vi "期末專題_PlantFactory Eleccost Calculator.vi"() -> ()   [LabVIEW 2014]
panel:
  in  "PlantFactory Eleccost Calculator":T1
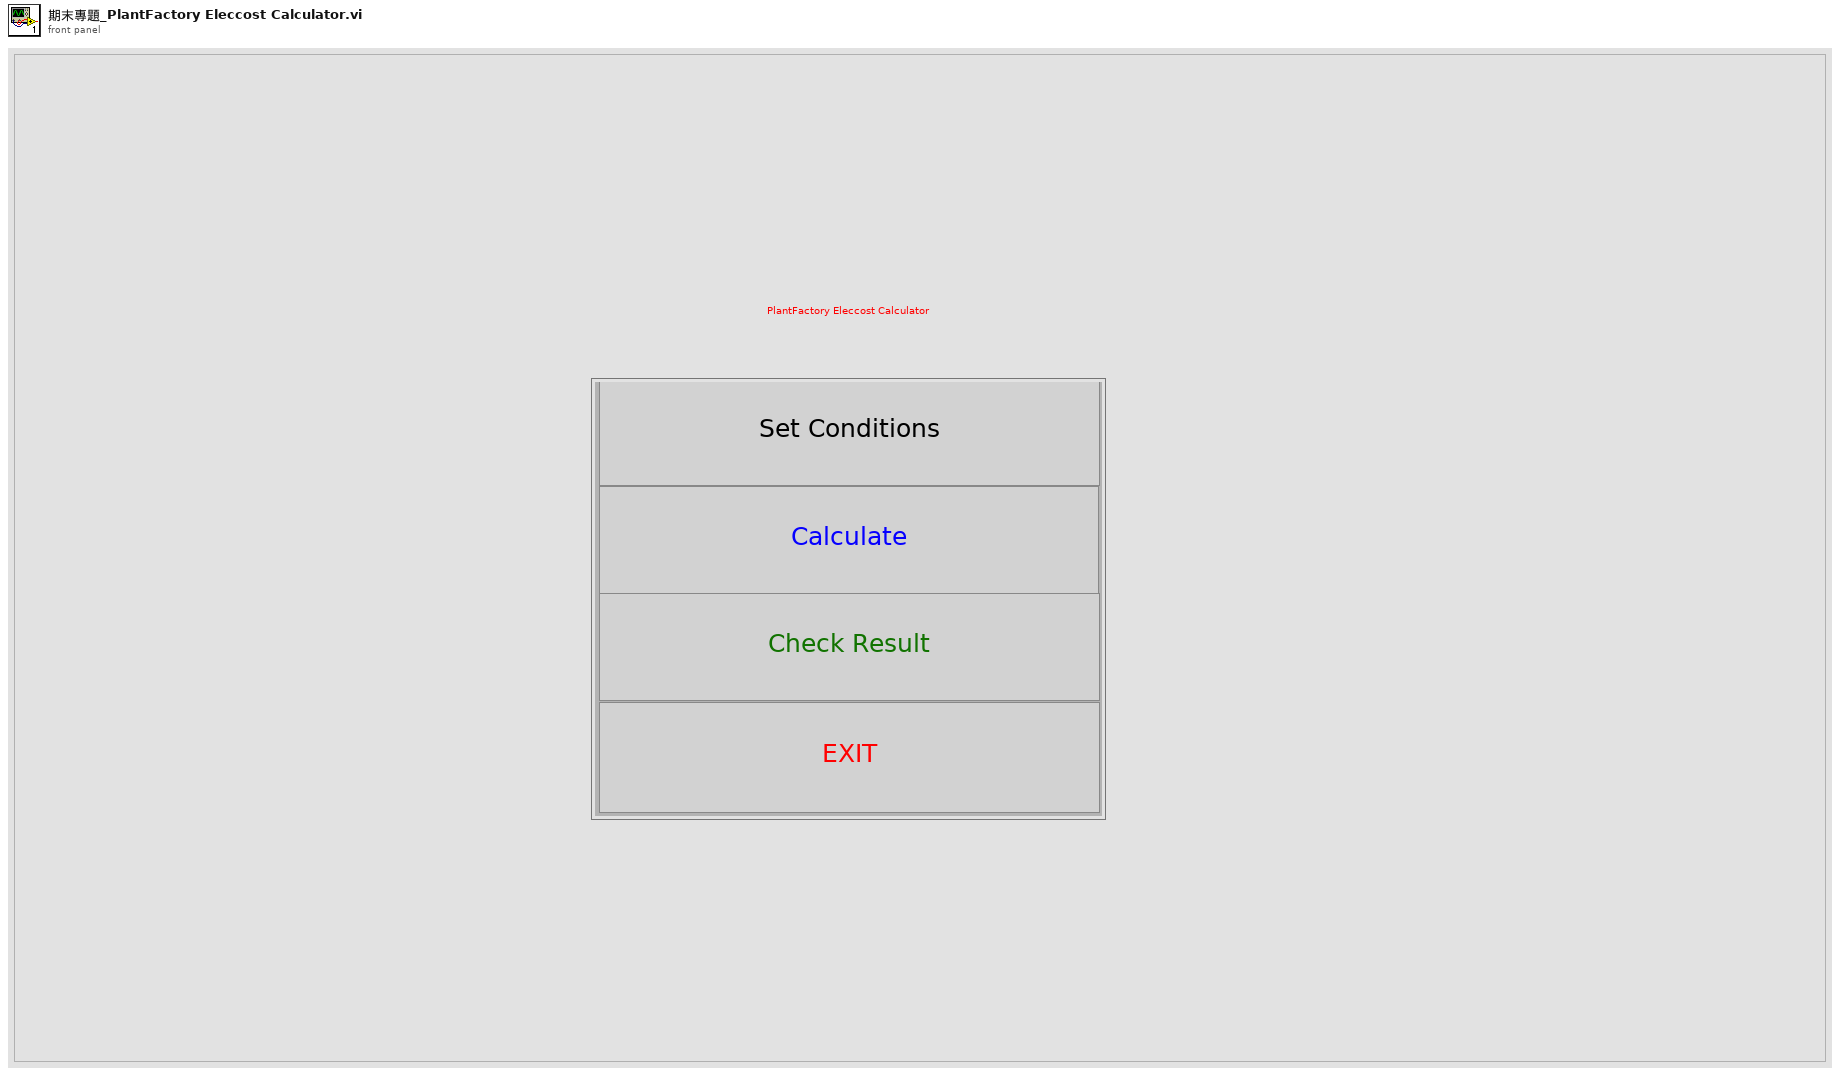
[diagram p1: front panel]
types:
  T1 = cluster{"set condi":bool, "calcu":bool, "outcome":bool, "exit":bool}
  T2 = cluster{"group Outcome":cluster{"Lightening Schedule":bool[], "group hourly total elecFee":dbl[], "group Total elecFee":dbl, "group hourly ACs elecFee":dbl[], "group ACs elecFee":dbl, "group hourly LEDs elecFee":dbl[], "group Total LEDs elecFee":dbl}, "group Outcome 2":cluster{"Lightening Schedule":bool[], "group hourly total elecFee":dbl[], "group Total elecFee":dbl, "group hourly ACs elecFee":dbl[], "group ACs elecFee":dbl, "group hourly LEDs elecFee":dbl[], "group Total LEDs elecFee":dbl}, "group Outcome 3":cluster{"Lightening Schedule":bool[], "group hourly total elecFee":dbl[], "group Total elecFee":dbl, "group hourly ACs elecFee":dbl[], "group ACs elecFee":dbl, "group hourly LEDs elecFee":dbl[], "group Total LEDs elecFee":dbl}, "Total elecFee":dbl}[]
  T3 = cluster{"input COP of ACs":dbl, "input setDay Temp":dbl, "input setNight Temp.":dbl}
  T4 = enum16{"wait button pressed", "init", "set conditions", "calcu", " outcome display"}
  T5 = enum8{"Enabled", "Disabled", "Disabled and Grayed Out"}
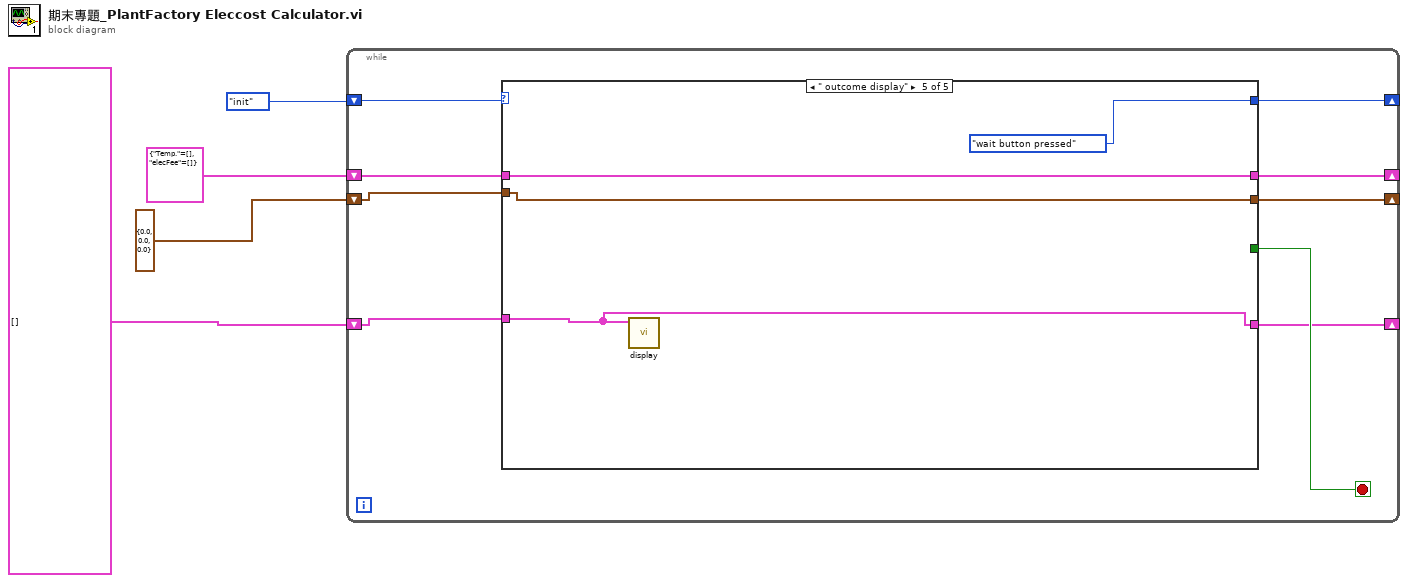
[diagram p0: block diagram]
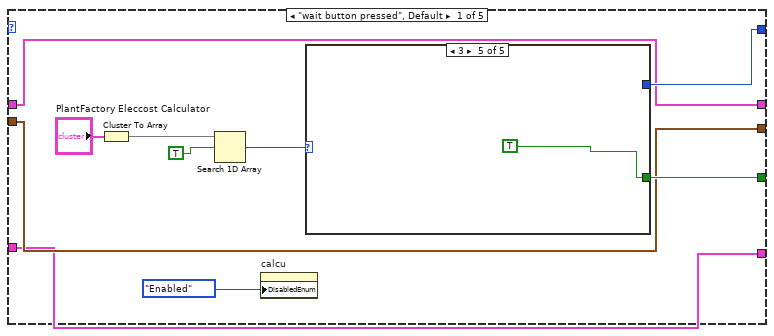
[diagram p2: hidden frame]
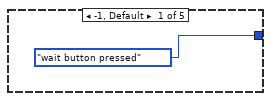
[diagram p3: hidden frame]
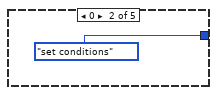
[diagram p4: hidden frame]
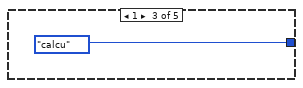
[diagram p5: hidden frame]
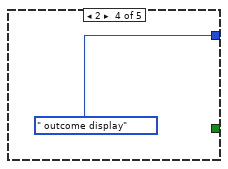
[diagram p6: hidden frame]
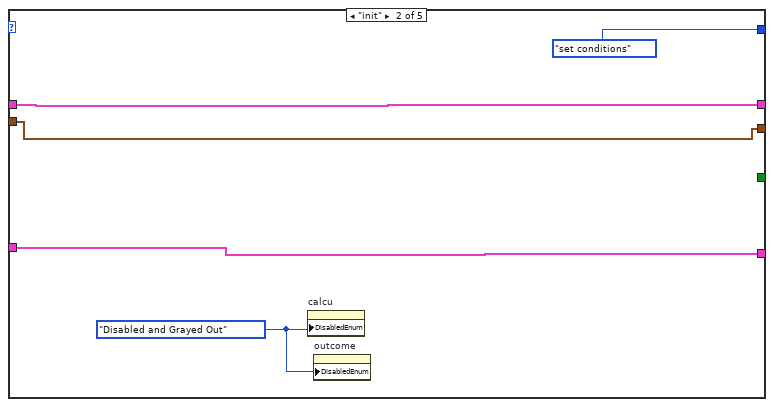
[diagram p7: hidden frame]
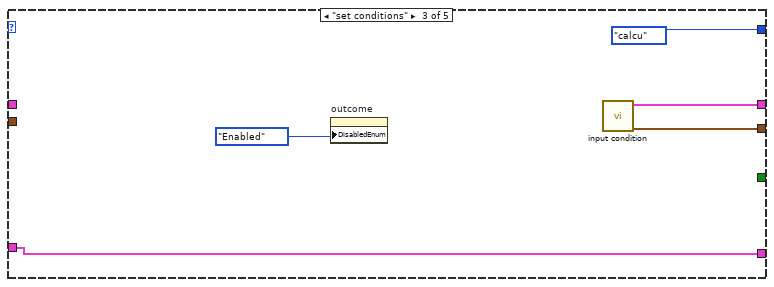
[diagram p8: hidden frame]
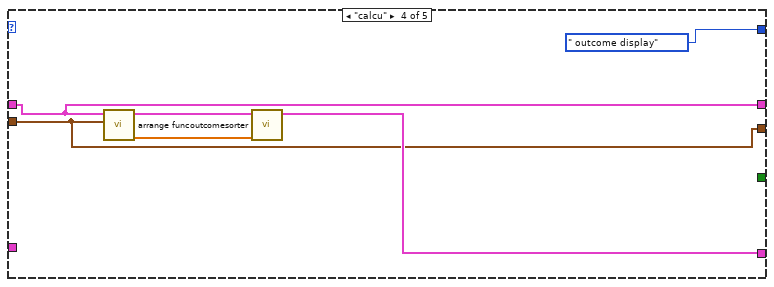
[diagram p9: hidden frame]
diagram:
  n1 = while {
    shift-right: [w13] -> _
    shift-left: T4."init" -> [w12]
    shift-right: [w10] -> _
    shift-left: cluster{"Temp.":dbl[], "elecFee":dbl[]} {"Temp."=[], "elecFee"=[]} ("input envTemp. & elecFee 2") -> [w7]
    shift-right: [w9] -> _
    shift-left: T3 {"input COP of ACs"=0.0, "input setDay Temp"=0.0, "input setNight Temp."=0.0} ("input Parameter 2") -> [w8]
    shift-right: [w6] -> _
    shift-left: T2 [] ("sorted Outcome") -> [w5]
    stop <- w11 stop-if-true
    n2 = case shown="\" outcome display\"" w12 {
      tunnel: [w18 T4."set conditions" T4."calcu" T4." outcome display" T4."wait button pressed"] -> w13
      tunnel: [w17 _ _ _ _] -> w11
      tunnel: [w16 w31 w38 w40 w47] -> w10
      tunnel: [w15 w30 w37 w39 w46] -> w9
      tunnel: w8 -> [w15 w30 _ w39 w46]
      tunnel: w7 -> [w16 w31 _ w40 w47]
      tunnel: [w14 w29 w34 w42 w45] -> w6
      tunnel: w5 -> [w14 w29 w34 _ w45]
      frame "wait button pressed", Default {
        n3 = Cluster To Array(cluster="PlantFactory Eleccost Calculator") -> (array=w22:bool[])
        n4 = Search 1D Array(1D array=w22, element=TRUE) -> (index of element=w19:i32)  [unwired: 1 in]
        n5 = property on="calcu" class="Bool"("DisabledEnum"=T5."Enabled" ("Disabled")) -> ()  [unwired: 2 in, 2 out]
        n6 = case shown="3" w19 {
          tunnel: [T4."wait button pressed" T4."set conditions" T4."calcu" T4." outcome display" _] -> w18
          tunnel: [_ _ _ _ TRUE] -> w17
          frame -1, Default {
          }
          frame 0 {
          }
          frame 1 {
          }
          frame 2 {
          }
          frame 3 {
          }
        }
      }
      frame "init" {
        w33 = T5."Disabled and Grayed Out" ("Disabled")
        n7 = property on="calcu" class="Bool"("DisabledEnum"=w33) -> ()  [unwired: 2 in, 2 out]
        n8 = property on="outcome" class="Bool"("DisabledEnum"=w33) -> ()  [unwired: 2 in, 2 out]
      }
      frame "set conditions" {
        n9 = property on="outcome" class="Bool"("DisabledEnum"=T5."Enabled" ("Disabled")) -> ()  [unwired: 2 in, 2 out]
        n10 = call "input condition.vi"() -> ("input Parameter 2"=w37:T3, "input envTemp. & elecFee 2"=w38:cluster{"Temp.":dbl[], "elecFee":dbl[]})  [unwired: 10 in]
      }
      frame "calcu" {
        n11 = call "arrange func.vi"("input Parameter"=w39, "input envTemp. & elecFee"=w40) -> ("Outcome Total elecFee"=w43:dbl[], "OUTCOME"=w44:T2)  [unwired: 8 in]
        n12 = call "outcomesorter.vi"("Outcome Total elecFee"=w43, "OUTCOME"=w44) -> ("sorted Outcome"=w42:T2)  [unwired: 9 in]
      }
      frame " outcome display" {
        n13 = call "display.vi"("Array"=w45) -> ()  [unwired: 11 in]
      }
    }
  }
